vi "UHR-Fleezers Control (host) - Avogadro v1.vi"() -> ()   [LabVIEW 2014] (continued)
        n65 = event-data() -> ()  [unwired: 1 in, 5 out]
        n66 = Build Array("Set Position 1", "Set Position 2", "Set Position 3", "Set Position 4", "Set Position 5", "Set Position 6") -> (w238:bool[])
        n67 = Boolean Array To Number(Boolean array=w238) -> (number=w237:u32)
        n68 = Logarithm Base 2(1:w237) -> (0:w229:dbl)
        n69 = call "Read Stage Position.vi"("error in"=w239, "VISA resource name in"=w240) -> ("Current Position"=w244:cluster{dbl, dbl, dbl}, "error out"=w243:errorcluster)  [unwired: 2 out]
        n70 = Decrement(x="Position") -> (x-1=w227:dbl)
        n71 = Greater Or Equal?(x=w229, y=0.0) -> (x >= y?=w230:bool)
        n72 = Cluster To Array(cluster=w244) -> (array=w241:dbl[])
        n73 = Select(t=w229, s=w230, f=w227) -> (s? t:f=w226:dbl)
        n74 = local write "Stage Control Serial Error"(w243) -> ()
        n75 = Increment(x=w226) -> (x+1=w225:dbl)
        n76 = Build Array (concatenate)(w225, w241) -> (w224:dbl[])
        n77 = Replace Array Subset(array="Saved Stage Positions", new element=w224, index (row)=w226) -> (w242:dbl[][])  [unwired: 1 in]
        n78 = local write "Saved Stage Positions"(w242) -> ()
      }
      event Menu Selection (User) {
        n79 = event-data() -> ("ItemTag"=w249:string)  [unwired: 1 in, 6 out]
        n80 = case shown="\"Z\"" w249 {
          tunnel: w248 -> [_ w251 w256 _]
          tunnel: w247 -> [_ w250 w254 _]
          frame "False", Default {
          }
          frame "XY" {
            n81 = call "start_stage_trackball.vi"("Enum"=T38."Trackball XY", "error in (no error)"=w250, "Stage Controller port"=w251) -> ("error out"=w253:errorcluster)  [unwired: 1 out]
            n82 = property on="Stage Control Serial Error" class="Clust (strict)"("Val(Sgnl)"=w253) -> ()  [unwired: 2 in, 2 out]
          }
          frame "Z" {
            n83 = call "start_stage_trackball.vi"("Enum"=T38."Trackball Z", "error in (no error)"=w254, "Stage Controller port"=w256) -> ("error out"=w255:errorcluster)  [unwired: 1 out]
            n84 = property on="Stage Control Serial Error" class="Clust (strict)"("Val(Sgnl)"=w255) -> ()  [unwired: 2 in, 2 out]
          }
          frame "True" {
          }
        }
      }
      event "Move to Position": Value Change {
        n85 = event-data() -> ()  [unwired: 1 in, 5 out]
        n86 = flat-sequence {
          tunnel: w259 -> [w263]
          tunnel: w258 -> [w262]
          frame #0 {
            n87 = local read "Saved Stage Positions"() -> (w265:dbl[][])
            n88 = local read "Position"() -> (w264:dbl)
            n89 = local write "Stage Moving"(TRUE ("Stage Moving")) -> ()
            n90 = call "move to saved stage position.vi"("error in"=w262, "Stage VISA resource name in"=w263, "Position"=w264, "Saved Stage Positions"=w265) -> ("error out"=w261:errorcluster)  [unwired: 1 out]
            n91 = local write "Stage Control Serial Error"(w261) -> ()
          }
          frame #1 {
            n92 = call <vilib>:"Beep.vi"() -> ()  [unwired: 3 in, 9 out]
            n93 = local write "Stage Moving"(FALSE ("Stage Moving")) -> ()
          }
        }
      }
      event "Move Cap. 1 (DNA Bottom)": Value Change {
        n94 = event-data() -> ()  [unwired: 1 in, 5 out]
        n95 = local write "Move Cap. 1 (DNA Bottom)"(FALSE ("Move Cap. 1 (DNA Right)")) -> ()
        n96 = flat-sequence {
          tunnel: w271 -> [w274]
          tunnel: w272 -> [w275]
          tunnel: [w275] -> w269
          tunnel: [w274] -> w268
          tunnel: w269 -> [w277]
          tunnel: w268 -> [w276]
          frame #0 {
            n97 = property on="Sample Channel\nFlow" class="Bool (strict)"("Val(Sgnl)"="Cap 1 Samp Flow ON") -> ()  [unwired: 2 in, 2 out]
          }
          frame #1 {
            n98 = local read "Saved Stage Positions"() -> (w287:dbl[][])
            n99 = local write "Stage Moving"(TRUE ("Stage Moving")) -> ()
            n100 = Array Subset(array=w287, index (row)=0 ("index"), length (row)=1 ("length"), index (col)=1 ("index"), length (col)=3 ("length")) -> (w284:dbl[][])
            n101 = Reshape Array(w284, 3 ("dimension size")) -> (w282:dbl[])
            n102 = Array To Cluster(array=w282) -> (cluster=w281:cluster{"[0]":dbl, "[1]":dbl, "[2]":dbl})
            n103 = call "Set Stage Position.vi"("Position"=w281, "error in"=w276, "VISA resource name in"=w277) -> ("error out"=w280:errorcluster)  [unwired: 2 out]
            n104 = local write "Stage Control Serial Error"(w280) -> ()
          }
          frame #2 {
            n105 = local write "Stage Moving"(FALSE ("Stage Moving")) -> ()
            n106 = case shown="True" "Cap 1 Flow ON" {
              frame False {
              }
              frame True {
                n107 = property on="Inject Pump 1" class="Bool (strict)"("Val(Sgnl)"=TRUE ("Value (Signaling)")) -> ()  [unwired: 2 in, 2 out]
              }
            }
            n108 = call <vilib>:"Beep.vi"() -> ()  [unwired: 3 in, 9 out]
          }
          frame #3 {
            n109 = property on="Sample Channel\nFlow" class="Bool (strict)"("Val(Sgnl)"=FALSE ("Value (Signaling)")) -> ()  [unwired: 2 in, 2 out]
            n110 = local read "Cap. 2 BD T1?\n(ADig T1, DNA T2)"() -> (w294:bool)
            n111 = case shown="True" w294 {
              tunnel: "Cap 1 T ON" -> [w296 w297]
              frame False {
                n112 = property on="Trap 1 (ON/OFF)" class="Bool (strict)"("Val(Sgnl)"=w296) -> ()  [unwired: 2 in, 2 out]
              }
              frame True {
                n113 = property on="Trap 2 (ON/OFF)" class="Bool (strict)"("Val(Sgnl)"=w297) -> ()  [unwired: 2 in, 2 out]
              }
            }
            n114 = property on="Get bead 2" class="Bool (strict)"("Key Focus"=TRUE) -> ()  [unwired: 2 in, 2 out]
          }
        }
      }
      event "Move Cap. 2 (ADig Top)": Value Change {
        n115 = event-data() -> ()  [unwired: 1 in, 5 out]
        n116 = local write "Move Cap. 2 (ADig Top)"(FALSE ("Move Cap. 2 (ADig Left)")) -> ()
        n117 = flat-sequence {
          tunnel: w301 -> [w304]
          tunnel: w302 -> [w305]
          tunnel: [w305] -> w299
          tunnel: [w304] -> w298
          tunnel: w299 -> [w308]
          tunnel: w298 -> [w307]
          frame #0 {
            n118 = property on="Sample Channel\nFlow" class="Bool (strict)"("Val(Sgnl)"="Cap 2 Samp Flow ON") -> ()  [unwired: 2 in, 2 out]
          }
          frame #1 {
            w306 = FALSE ("Value (Signaling)")
            n119 = local read "Saved Stage Positions"() -> (w318:dbl[][])
            n120 = local write "Stage Moving"(TRUE ("Stage Moving")) -> ()
            n121 = Array Subset(array=w318, index (row)=1 ("index"), length (row)=1 ("length"), index (col)=1 ("index"), length (col)=3 ("length")) -> (w315:dbl[][])
            n122 = Reshape Array(w315, 3 ("dimension size")) -> (w313:dbl[])
            n123 = property on="Trap 1 (ON/OFF)" class="Bool (strict)"("Val(Sgnl)"=w306) -> ()  [unwired: 2 in, 2 out]
            n124 = property on="Trap 1 (ON/OFF)" class="Bool (strict)"("Val(Sgnl)"=w306) -> ()  [unwired: 2 in, 2 out]
            n125 = Array To Cluster(array=w313) -> (cluster=w312:cluster{"[0]":dbl, "[1]":dbl, "[2]":dbl})
            n126 = call "Set Stage Position.vi"("Position"=w312, "error in"=w307, "VISA resource name in"=w308) -> ("error out"=w311:errorcluster)  [unwired: 2 out]
            n127 = local write "Stage Control Serial Error"(w311) -> ()
          }
          frame #2 {
            n128 = local write "Stage Moving"(FALSE ("Stage Moving")) -> ()
            n129 = call <vilib>:"Beep.vi"() -> ()  [unwired: 3 in, 9 out]
            n130 = case shown="True" "Cap 2 Flow ON" {
              frame False {
              }
              frame True {
                n131 = property on="Inject Pump 3" class="Bool (strict)"("Val(Sgnl)"=TRUE ("Value (Signaling)")) -> ()  [unwired: 2 in, 2 out]
              }
            }
          }
          frame #3 {
            n132 = property on="Sample Channel\nFlow" class="Bool (strict)"("Val(Sgnl)"=FALSE ("Value (Signaling)")) -> ()  [unwired: 2 in, 2 out]
            n133 = case shown="False" "Cap. 2 BD T1?\n(ADig T1, DNA T2)" {
              tunnel: "Cap 2 T ON" -> [w327 w328]
              frame False {
                n134 = property on="Trap 2 (ON/OFF)" class="Bool (strict)"("Val(Sgnl)"=w327) -> ()  [unwired: 2 in, 2 out]
              }
              frame True {
                n135 = property on="Trap 1 (ON/OFF)" class="Bool (strict)"("Val(Sgnl)"=w328) -> ()  [unwired: 2 in, 2 out]
              }
            }
            n136 = property on="Get bead 3" class="Bool (strict)"("Key Focus"=TRUE) -> ()  [unwired: 2 in, 2 out]
          }
        }
      }
      event "Send string\nto Blue Laser": Value Change {
        n137 = event-data() -> ()  [unwired: 1 in, 5 out]
        n138 = flat-sequence {
          tunnel: w329 -> [w330]
          frame #0 {
            n139 = call "serial write macro.vi"("String"="command string", "Delay (ms)"="Delay (ms)", "VISA resource name"=w330) -> ("read buffer"=→"read blue buffer":string, "error out"=→"Blue Error Out":errorcluster)  [unwired: 1 out]
            "command string sent" <- "command string"
          }
          frame #1 {
            n140 = local write "Send string\nto Blue Laser"(FALSE ("Send string")) -> ()
          }
        }
      }
      event "Get Blue Laser State": Value Change {
        n141 = event-data() -> ()  [unwired: 1 in, 5 out]
        n142 = local read "Delay (ms)"() -> (w337:i32)
        n143 = flat-sequence {
          tunnel: w337 -> [w345]
          tunnel: w336 -> [w348]
          tunnel: [w346] -> w341
          tunnel: [w345] -> w340
          tunnel: [w355] -> w339
          tunnel: [w352] -> w338
          tunnel: w341 -> [w353]
          tunnel: w340 -> [w352]
          tunnel: w339 -> [w361]
          tunnel: w338 -> [w359]
          frame #0 {
            w343 = "l?"
            n144 = local write "command string sent"(w343) -> ()
            n145 = call "serial write macro.vi"("String"=w343, "Delay (ms)"=w345, "VISA resource name"=w348) -> ("read buffer"=w344:string, "VISA resource name out"=w346:refnum<visa-resource-name>)  [unwired: 1 out]
            n146 = Decimal String To Number(string=w344) -> (number=w347:i32)  [unwired: 2 in, 1 out]
            n147 = Not Equal To 0?(x=w347) -> (x != 0?=→"Laser On":bool)
            n148 = local write "read blue buffer"(w344) -> ()
          }
          frame #1 {
            w350 = "games?" ("String")
            n149 = local write "command string sent"(w350) -> ()
            n150 = call "serial write macro.vi"("String"=w350, "Delay (ms)"=w352, "VISA resource name"=w353) -> ("read buffer"=w351:string, "VISA resource name out"=w355:refnum<visa-resource-name>)  [unwired: 1 out]
            n151 = Decimal String To Number(string=w351) -> (number=w354:i32)  [unwired: 2 in, 1 out]
            n152 = local write "read blue buffer"(w351) -> ()
            n153 = Not Equal To 0?(x=w354) -> (x != 0?=→"Analog Modulation":bool)
          }
          frame #2 {
            w357 = "gdmes?" ("String")
            n154 = local write "command string sent"(w357) -> ()
            n155 = call "serial write macro.vi"("String"=w357, "Delay (ms)"=w359, "VISA resource name"=w361) -> ("read buffer"=w358:string)  [unwired: 2 out]
            n156 = Decimal String To Number(string=w358) -> (number=w360:i32)  [unwired: 2 in, 1 out]
            n157 = Not Equal To 0?(x=w360) -> (x != 0?=→"Digital Modulation":bool)
            n158 = local write "read blue buffer"(w358) -> ()
          }
          frame #3 {
            n159 = local write "Get Blue Laser State"(FALSE) -> ()
          }
        }
      }
      event "Blue Laser Power (mW)\n(Constant Power Mode)", "Blue Laser Modulation\nPower (mW)": Value Change {
        n160 = event-data() -> ()  [unwired: 1 in, 5 out]
        n161 = flat-sequence {
          tunnel: w364 -> [w370]
          tunnel: [w368] -> w363
          tunnel: w363 -> [w377]
          frame #0 {
            n162 = local read "Delay (ms)"() -> (w369:i32)
            n163 = Concatenate Strings("slmp " ("string"), "Blue Laser Modulation\nPower (mW)") -> (w365:string)
            n164 = call "serial write macro.vi"("String"=w365, "Delay (ms)"=w369, "VISA resource name"=w370) -> ("read buffer"=w366:string, "error out"=w367:errorcluster, "VISA resource name out"=w368:refnum<visa-resource-name>)
            n165 = local write "command string sent"(w365) -> ()
            n166 = local write "read blue buffer"(w366) -> ()
            n167 = local write "Blue Error Out"(w367) -> ()
          }
          frame #1 {
            n168 = local read "Delay (ms)"() -> (w376:i32)
            n169 = Concatenate Strings("p " ("string"), "Blue Laser Power (mW)\n(Constant Power Mode)") -> (w373:string)
            n170 = call "serial write macro.vi"("String"=w373, "Delay (ms)"=w376, "VISA resource name"=w377) -> ("read buffer"=w374:string, "error out"=w375:errorcluster)  [unwired: 1 out]
            n171 = local write "command string sent"(w373) -> ()
            n172 = local write "read blue buffer"(w374) -> ()
            n173 = local write "Blue Error Out"(w375) -> ()
          }
        }
      }
      event "Laser interlacing mode", "Blue Laser Modulation Mode", "Blue Laser ON": Value Change {
        n174 = event-data() -> ()  [unwired: 1 in, 5 out]
        n175 = flat-sequence {
          tunnel: w383 -> [w388]
          tunnel: [w387] -> w380
          tunnel: [w393] -> w382
          tunnel: w380 -> [w396]
          tunnel: w382 -> [w408]
          tunnel: [w402] -> w381
          tunnel: w381 -> [w415]
          frame #0 {
            n176 = local read "Blue Laser ON"() -> (w385:bool)
            n177 = local read "Delay (ms)"() -> (w386:i32)
            n178 = case shown="False" w385 {
              tunnel: ["l0" "l1"] -> w384
              frame False {
              }
              frame True {
              }
            }
            n179 = call "serial write macro.vi"("String"=w384, "Delay (ms)"=w386, "VISA resource name"=w388) -> ("error out"=w389:errorcluster, "VISA resource name out"=w387:refnum<visa-resource-name>)  [unwired: 1 out]
            n180 = local write "Blue Error Out"(w389) -> ()
          }
          frame #1 {
            n181 = local read "Laser interlacing mode"() -> (w398:enum32{"Laser ON", "Laser OFF", "Interlace"})
            n182 = case shown="\"Laser ON\"" w398 {
              tunnel: ["cp" "em" "l0"] -> w392
              frame "Laser ON" {
              }
              frame "Interlace" {
              }
              frame "Laser OFF", Default {
              }
            }
            n183 = local read "Delay (ms)"() -> (w397:i32)
            n184 = call "serial write macro.vi"("String"=w392, "Delay (ms)"=w397, "VISA resource name"=w396) -> ("read buffer"=w394:string, "error out"=w395:errorcluster, "VISA resource name out"=w393:refnum<visa-resource-name>)
            n185 = local write "command string sent"(w392) -> ()
            n186 = local write "read blue buffer"(w394) -> ()
            n187 = local write "Blue Error Out"(w395) -> ()
          }
          frame #2 {
            n188 = case shown="\"Analog Modulation\"" "Blue Laser Modulation Mode" {
              tunnel: ["sdmes 0" "sdmes 1" "sdmes 1"] -> w403
              frame "Analog Modulation" {
              }
              frame "Digital + Analog Modulation" {
              }
              frame "Digital Modulation", Default {
              }
            }
            n189 = local read "Delay (ms)"() -> (w406:i32)
            n190 = call "serial write macro.vi"("String"=w403, "Delay (ms)"=w406, "VISA resource name"=w408) -> ("read buffer"=w404:string, "error out"=w405:errorcluster, "VISA resource name out"=w402:refnum<visa-resource-name>)
            n191 = local write "command string sent"(w403) -> ()
            n192 = local write "read blue buffer"(w404) -> ()
            n193 = local write "Blue Error Out"(w405) -> ()
          }
          frame #3 {
            n194 = local read "Blue Laser Modulation Mode"() -> (w417:string)
            n195 = case shown="\"Digital Modulation\", Default" w417 {
              tunnel: ["sames 1" "sames 1" "sames 0"] -> w413
              frame "Analog Modulation" {
              }
              frame "Digital + Analog Modulation" {
              }
              frame "Digital Modulation", Default {
              }
            }
            n196 = local read "Delay (ms)"() -> (w416:i32)
            n197 = local write "command string sent"(w413) -> ()
            n198 = call "serial write macro.vi"("String"=w413, "Delay (ms)"=w416, "VISA resource name"=w415) -> ("read buffer"=w414:string, "error out"=w412:errorcluster)  [unwired: 1 out]
            n199 = local write "read blue buffer"(w414) -> ()
            n200 = local write "Blue Error Out"(w412) -> ()
          }
        }
      }
      event "Read Harvard": Value Change {
        n201 = event-data() -> ()  [unwired: 1 in, 5 out]
        n202 = Concatenate Strings("write buffer", "\r") -> (w425:string)
        n203 = VISA Write(VISA resource name=w423, write buffer=w425, error in (no error)=w422) -> (VISA resource name out=w434:refnum<visa-resource-name>, error out=w433:errorcluster)  [unwired: 1 out]
        n204 = stacked-sequence {
          tunnel: [w437] -> w432
          tunnel: w434 -> [w437]
          tunnel: w433 -> [w436]
          tunnel: [w436] -> w427
          frame #0 {
            n205 = Wait (ms)(milliseconds to wait=50) -> ()  [unwired: 1 out]
          }
        }
        n206 = property class="Instr"(reference=w432, error in=w427) -> (reference out=w431:refnum<visa-resource-name>, error out=w429:errorcluster, "Serial Settings:Number of Bytes at Serial Port"=w430:u32)
        "Serial Settings:Number of Bytes at Serial Port" <- w430
        n207 = VISA Read(VISA resource name=w431, byte count=w430, error in (no error)=w429) -> (read buffer=w428:string)  [unwired: 3 out]
        "read buffer" <- w428
        n208 = Fract/Exp String To Number(string=w428) -> ()  [unwired: 5 out]
      }
      event "+z", "-z": Value Change {
        n209 = event-data() -> ()  [unwired: 1 in, 5 out]
        n210 = flat-sequence {
          tunnel: w438 -> [w460]
          tunnel: w439 -> [w440]
          frame #0 {
            n211 = call "Read Stage Position.vi"("error in"=w460, "VISA resource name in"=w440) -> ("Current Position"=w445:cluster{dbl, dbl, dbl}, "error out"=w458:errorcluster, "VISA resource name out"=w459:refnum<visa-resource-name>)  [unwired: 1 out]
            n212 = local read "Saved Stage Positions"() -> (w469:dbl[][])
            n213 = Divide(x="z nudge increment (um)", y=1000.0) -> (x/y=w457:dbl)
            n214 = Boolean To (0,1)(Boolean="+z") -> (0, 1=w449:i16)
            n215 = Boolean To (0,1)(Boolean="-z") -> (0, 1=w450:i16)
            n216 = Array Subset(array=w469, index (row)=1 ("index"), length (row)=1 ("length"), index (col)=1 ("index"), length (col)=3 ("length")) -> (w466:dbl[][])
            n217 = Multiply(x=w449, y=w457) -> (x*y=w453:dbl)
            n218 = Multiply(x=w450, y=w457) -> (x*y=w451:dbl)
            n219 = Unbundle(w445) -> (w443:dbl, w442:dbl, w446:dbl)
            n220 = Negate(x=w451) -> (-x=w452:dbl)
            n221 = Reshape Array(w466, 3 ("dimension size")) -> (w464:dbl[])
            n222 = Add(x=w453, y=w452) -> (x+y=w454:dbl)
            n223 = Array To Cluster(array=w464) -> ()  [unwired: 1 out]
            n224 = Add(x=w454, y=w446) -> (x+y=w444:dbl)
            n225 = Bundle(cluster=w445, w443, w442, w444) -> (w441:cluster{dbl, dbl, dbl})
            n226 = call "Set Stage Position.vi"("Position"=w441, "error in"=w458, "VISA resource name in"=w459) -> ("error out"=w463:errorcluster)  [unwired: 2 out]
            n227 = local write "Stage Moving"(TRUE ("Stage Moving")) -> ()
            n228 = local write "Stage Control Serial Error"(w463) -> ()
          }
          frame #1 {
            n229 = local write "Stage Moving"(FALSE ("Stage Moving")) -> ()
          }
        }
      }
      event "-y", "+y": Value Change {
        n230 = event-data() -> ()  [unwired: 1 in, 5 out]
        n231 = flat-sequence {
          tunnel: w472 -> [w496]
          tunnel: w473 -> [w479]
          frame #0 {
            n232 = call "Read Stage Position.vi"("error in"=w496, "VISA resource name in"=w479) -> ("Current Position"=w482:cluster{dbl, dbl, dbl}, "error out"=w494:errorcluster, "VISA resource name out"=w495:refnum<visa-resource-name>)  [unwired: 1 out]
            n233 = Divide(x="y nudge increment (um", y=1000.0) -> (x/y=w493:dbl)
            n234 = Boolean To (0,1)(Boolean="+y") -> (0, 1=w485:i16)
            n235 = Boolean To (0,1)(Boolean="-y") -> (0, 1=w486:i16)
            n236 = Multiply(x=w485, y=w493) -> (x*y=w489:dbl)
            n237 = Multiply(x=w486, y=w493) -> (x*y=w487:dbl)
            n238 = Unbundle(w482) -> (w481:dbl, w476:dbl, w478:dbl)
            n239 = Negate(x=w487) -> (-x=w488:dbl)
            n240 = Add(x=w489, y=w488) -> (x+y=w490:dbl)
            n241 = Add(x=w490, y=w476) -> (x+y=w477:dbl)
            n242 = Bundle(cluster=w482, w481, w477, w478) -> (w480:cluster{dbl, dbl, dbl})
            n243 = call "Set Stage Position.vi"("Position"=w480, "error in"=w494, "VISA resource name in"=w495) -> ("error out"=w475:errorcluster)  [unwired: 2 out]
            n244 = local write "Stage Control Serial Error"(w475) -> ()
            n245 = local write "Stage Moving"(TRUE ("Stage Moving")) -> ()
          }
          frame #1 {
            n246 = local write "Stage Moving"(FALSE ("Stage Moving")) -> ()
          }
        }
      }
      event "-x", "+x": Value Change {
        n247 = event-data() -> ()  [unwired: 1 in, 5 out]
        n248 = flat-sequence {
          tunnel: w498 -> [w522]
          tunnel: w499 -> [w506]
          frame #0 {
            n249 = call "Read Stage Position.vi"("error in"=w522, "VISA resource name in"=w506) -> ("Current Position"=w508:cluster{dbl, dbl, dbl}, "error out"=w520:errorcluster, "VISA resource name out"=w521:refnum<visa-resource-name>)  [unwired: 1 out]
            n250 = Divide(x="x nudge increment (um)", y=1000.0) -> (x/y=w519:dbl)
            n251 = Boolean To (0,1)(Boolean="+x") -> (0, 1=w511:i16)
            n252 = Boolean To (0,1)(Boolean="-x") -> (0, 1=w512:i16)
            n253 = Multiply(x=w511, y=w519) -> (x*y=w515:dbl)
            n254 = Multiply(x=w512, y=w519) -> (x*y=w513:dbl)
            n255 = Unbundle(w508) -> (w500:dbl, w502:dbl, w505:dbl)
            n256 = Negate(x=w513) -> (-x=w514:dbl)
            n257 = Add(x=w515, y=w514) -> (x+y=w516:dbl)
            n258 = Add(x=w516, y=w500) -> (x+y=w501:dbl)
            n259 = Bundle(cluster=w508, w501, w502, w505) -> (w507:cluster{dbl, dbl, dbl})
            n260 = call "Set Stage Position.vi"("Position"=w507, "error in"=w520, "VISA resource name in"=w521) -> ("error out"=w503:errorcluster)  [unwired: 2 out]
            n261 = local write "Stage Control Serial Error"(w503) -> ()
            n262 = local write "Stage Moving"(TRUE ("Stage Moving")) -> ()
          }
          frame #1 {
            n263 = local write "Stage Moving"(FALSE ("Stage Moving")) -> ()
          }
        }
      }
      event "Cal/Data Acq. Spot": Value Change {
        # "03-01-2018 Changed by RG to incorporate offset measurements at multiple \npositions of the piezo mirror"
        # "Disabled by Ronen - we have our own way of controlling the location of calibration."
        n264 = event-data() -> ()  [unwired: 1 in, 5 out]
        n265 = flat-sequence {
          tunnel: w531 -> [w535]
          tunnel: w532 -> [w536]
          tunnel: [w536] -> w528
          tunnel: [w535] -> w527
          tunnel: w528 -> [w539]
          tunnel: w527 -> [w538]
          tunnel: ["Cal @ (MHz)"] -> w525
          tunnel: [w547] -> w529
          tunnel: w525 -> [w547]
          tunnel: w529 -> [w560]
          tunnel: ["W/ Offset 1"] -> w526
          tunnel: w524 -> [w558]
          tunnel: w529 -> [w596]
          tunnel: w526 -> [w594]
          frame #0 {
            n266 = property on="Sample Channel\nFlow" class="Bool (strict)"("Val(Sgnl)"="Daq spot flow on") -> ()  [unwired: 2 in, 2 out]
            n267 = Wait (ms)(milliseconds to wait=u32 250) -> ()  [unwired: 1 out]
          }
          frame #1 {
            n268 = disable-structure shown="Disabled" {
              disable-tunnel: w539 -> [w544 _]
              disable-tunnel: w538 -> [w543 _]
              frame Disabled {
                n269 = local read "Saved Stage Positions"() -> (w541:dbl[][])
                n270 = call "move to saved stage position.vi"("error in"=w543, "Stage VISA resource name in"=w544, "Position"="Cal Stage Position", "Saved Stage Positions"=w541) -> ("error out"=w542:errorcluster)  [unwired: 1 out]
                n271 = local write "Stage Control Serial Error"(w542) -> ()
              }
              frame Enabled {
              }
            }
            n272 = property on="Trap Delta (MHz)" class="DigNum (strict)"("Val(Sgnl)"="Cal @ (MHz)") -> ()  [unwired: 2 in, 2 out]
            n273 = local write "Stage Moving"(TRUE ("Stage Moving")) -> ()
          }
          frame #2 {
            n274 = local write "Stage Moving"(FALSE ("Stage Moving")) -> ()
            n275 = property on="Sample Channel\nFlow" class="Bool (strict)"("Val(Sgnl)"="Flow ON during cal?") -> ()  [unwired: 2 in, 2 out]
            n276 = call <vilib>:"Beep.vi"() -> ()  [unwired: 3 in, 9 out]
          }
          frame #3 {
            n277 = Wait (ms)(milliseconds to wait=u32 1000) -> ()  [unwired: 1 out]
          }
          frame #4 {
            n278 = case shown="False" "Active cal after cal?" {
              frame False {
              }
              frame True {
                n279 = local write "Active Cal"(TRUE ("Active Cal")) -> ()
                n280 = Wait (ms)(milliseconds to wait=u32 8000) -> ()  [unwired: 1 out]
              }
            }
          }
          frame #5 {
            n281 = property on="Save Calibration" class="Bool (strict)"("Val(Sgnl)"=TRUE ("Value (Signaling)")) -> ()  [unwired: 2 in, 2 out]
          }
          frame #6 {
            n282 = Wait (ms)(milliseconds to wait=u32 2000) -> ()  [unwired: 1 out]
          }
          frame #7 {
            # "Check to see if \nsaving done"
            n283 = while {
              stop <- w555 stop-if-true
              n284 = local read "Saving..."() -> (w556:bool)
              n285 = Wait (ms)(milliseconds to wait=u32 100) -> ()  [unwired: 1 out]
              n286 = Not(x=w556) -> (.not. x?=w555:bool)
            }
          }
          frame #8 {
            n287 = case shown="True" "W/ Offset 1" {
              tunnel: w560 -> [_ w562]
              tunnel: w558 -> [_ w561]
              frame False {
              }
              frame True {
                n288 = stacked-sequence {
                  tunnel: w562 -> [_ _ _ _ _ _ _ _ _ w593]
                  tunnel: w561 -> [_ _ _ _ w571 _ _ _ _ w591]
                  frame #0 {
                    n289 = property on="Trap Delta (MHz)" class="DigNum (strict)"("Val(Sgnl)"="Offset 1 Start (MHz)") -> ()  [unwired: 2 in, 2 out]
                    n290 = Replace Array Subset(array=u32[] [0] ("Index Values"), new element="Offset 1 Set", index=0) -> (w564:u32[])
                    n291 = property on="Saved AOD Raster Scan Parameter Sets" class="Arr (strict)"("Index Values"=w564) -> ()  [unwired: 2 in, 2 out]
                    n292 = property on="manual raster set" class="Ring (strict)"("Value"="Offset 1 Set") -> ()  [unwired: 2 in, 2 out]
                  }
                  frame #1 {
                    n293 = Wait (ms)(milliseconds to wait=u32 200) -> ()  [unwired: 1 out]
                  }
                  frame #2 {
                    n294 = property on="Load parameters" class="Bool (strict)"("Val(Sgnl)"=TRUE ("Value (Signaling)")) -> ()  [unwired: 2 in, 2 out]
                  }
                  frame #3 {
                    n295 = Wait (ms)(milliseconds to wait=u32 200) -> ()  [unwired: 1 out]
                  }
                  frame #4 {
                    n296 = case shown="True" "Multiple-MCL offset?" {
                      tunnel: w571 -> [_ w580]
                      frame False {
                      }
                      frame True {
                        n297 = call "Make Trap3 position array.vi"("MCL offset scanning range (V)"="MCL offset scanning range (V)") -> ("Scan increment"=w575:u64, "Min Y"=w576:u64, "Min X"=w577:u64, "X Data points"=w578:u64, "Y data points"=w579:u64)
                        n298 = Multiply(x=w579, y=w578) -> (x*y=w573:u64)
                        n299 = xnode "Read/Write Control"("FPGA VI Reference In"=w580, "Number of scans"=w573, "Piezo offset Y points"=w579, "Piezo offset X points"=w578, "Piezo offset Xmin"=w577, "Piezo Offset Ymin"=w576, "Piezo Offset Increment"=w575, "Multiple trap 3 position offset  file"=TRUE) -> ()  [unwired: 1 in, 2 out]
                        n300 = property on="Number of F/B Scans (AOD)" class="DigNum (strict)"("Val(Sgnl)"=w573) -> ()  [unwired: 2 in, 2 out]
                      }
                    }
                  }
                  frame #5 {
                    n301 = Wait (ms)(milliseconds to wait=u32 200) -> ()  [unwired: 1 out]
                  }
                  frame #6 {
                    n302 = property on="Trap Raster Scan" class="Bool (strict)"("Val(Sgnl)"=TRUE ("Value (Signaling)")) -> ()  [unwired: 2 in, 2 out]
                  }
                  frame #7 {
                    n303 = Wait (ms)(milliseconds to wait=u32 2000) -> ()  [unwired: 1 out]
                  }
                  frame #8 {
                    n304 = while {
                      stop <- w588 stop-if-true
                      n305 = local read "Raster Scanning..."() -> (w590:bool)
                      n306 = local read "Saving..."() -> (w586:bool)
                      n307 = Wait (ms)(milliseconds to wait=u32 100) -> ()  [unwired: 1 out]
                      n308 = Not(x=w586) -> (.not. x?=w585:bool)
                      n309 = Not(x=w590) -> (.not. x?=w587:bool)
                      n310 = And(x=w587, y=w585) -> (x .and. y?=w588:bool)
                    }
                  }
                  frame #9 {
                    n311 = property on="Trap Delta (MHz)" class="DigNum (strict)"("Val(Sgnl)"=w593) -> ()  [unwired: 2 in, 2 out]
                    n312 = xnode "Read/Write Control"("FPGA VI Reference In"=w591, "Multiple trap 3 position offset  file"=FALSE) -> ()  [unwired: 1 in, 2 out]
                  }
                }
              }
            }
          }
          frame #9 {
            n313 = local read "Save ave N"() -> (w595:dbl)
            n314 = case shown="False" "W/ Offset 2" {
              tunnel: w596 -> [_ w603]
              tunnel: w595 -> [_ w602]
              tunnel: w594 -> [w598 _]
              frame False {
                n315 = case shown="False" w598 {
                  frame False {
                    n316 = Multiply(x="Cal read wait (s)", y=u32 1000 ("milliseconds to wait")) -> (x*y=w600:u32)
                    n317 = Wait (ms)(milliseconds to wait=w600) -> ()  [unwired: 1 out]
                  }
                  frame True {
                  }
                }
              }
              frame True {
                n318 = stacked-sequence {
                  tunnel: w603 -> [_ _ _ _ _ _ _ _ _ w624 _ _]
                  tunnel: w602 -> [_ _ _ _ _ _ _ _ _ w622 _ _]
                  frame #0 {
                    n319 = property on="Save ave N" class="DigNum (strict)"("Val(Sgnl)"=1.0 ("Value (Signaling)")) -> ()  [unwired: 2 in, 2 out]
                  }
                  frame #1 {
                    n320 = Wait (ms)(milliseconds to wait=u32 500) -> ()  [unwired: 1 out]
                  }
                  frame #2 {
                    n321 = property on="Trap Delta (MHz)" class="DigNum (strict)"("Val(Sgnl)"="Offset 2 Start (MHz)") -> ()  [unwired: 2 in, 2 out]
                    n322 = Replace Array Subset(array=u32[] [0] ("Index Values"), new element="Offset 2 Set", index=0) -> (w608:u32[])
                    n323 = property on="Saved AOD Raster Scan Parameter Sets" class="Arr (strict)"("Index Values"=w608) -> ()  [unwired: 2 in, 2 out]
                  }
                  frame #3 {
                    n324 = Wait (ms)(milliseconds to wait=u32 500) -> ()  [unwired: 1 out]
                  }
                  frame #4 {
                    n325 = property on="Load parameters" class="Bool (strict)"("Val(Sgnl)"=TRUE ("Value (Signaling)")) -> ()  [unwired: 2 in, 2 out]
                  }
                  frame #5 {
                    n326 = Wait (ms)(milliseconds to wait=u32 500) -> ()  [unwired: 1 out]
                  }
                  frame #6 {
                    n327 = property on="Trap Raster Scan" class="Bool (strict)"("Val(Sgnl)"=TRUE ("Value (Signaling)")) -> ()  [unwired: 2 in, 2 out]
                  }
                  frame #7 {
                    n328 = Wait (ms)(milliseconds to wait=u32 2000) -> ()  [unwired: 1 out]
                  }
                  frame #8 {
                    n329 = while {
                      stop <- w617 stop-if-true
                      n330 = local read "Raster Scanning..."() -> (w620:bool)
                      n331 = local read "Saving..."() -> (w618:bool)
                      n332 = Wait (ms)(milliseconds to wait=u32 100) -> ()  [unwired: 1 out]
                      n333 = Not(x=w618) -> (.not. x?=w616:bool)
                      n334 = Not(x=w620) -> (.not. x?=w619:bool)
                      n335 = And(x=w619, y=w616) -> (x .and. y?=w617:bool)
                    }
                  }
                  frame #9 {
                    n336 = property on="Trap Delta (MHz)" class="DigNum (strict)"("Val(Sgnl)"=w624) -> ()  [unwired: 2 in, 2 out]
                    n337 = property on="Saved AOD Raster Scan Parameter Sets" class="Arr (strict)"("Index Values"=u32[] [0]) -> ()  [unwired: 2 in, 2 out]
                    n338 = property on="Save ave N" class="DigNum (strict)"("Val(Sgnl)"=w622) -> ()  [unwired: 2 in, 2 out]
                  }
                  frame #10 {
                    n339 = Wait (ms)(milliseconds to wait=u32 500) -> ()  [unwired: 1 out]
                  }
                  frame #11 {
                    n340 = property on="Load parameters" class="Bool (strict)"("Val(Sgnl)"=TRUE ("Value (Signaling)")) -> ()  [unwired: 2 in, 2 out]
                  }
                }
              }
            }
          }
          frame #10 {
            n341 = property on="Read Cal" class="Bool (strict)"("Val(Sgnl)"=TRUE ("Value (Signaling)")) -> ()  [unwired: 2 in, 2 out]
          }
          frame #11 {
            n342 = Wait (ms)(milliseconds to wait=u32 1000) -> ()  [unwired: 1 out]
          }
          frame #12 {
            n343 = property on="Fish for Tether" class="Bool (strict)"("Val(Sgnl)"="Fish after cal?") -> ()  [unwired: 2 in, 2 out]
          }
        }
        n344 = local write "Cal/Data Acq. Spot"(FALSE ("Cal/Data Acq. Spot")) -> ()
      }
      event "Dump Beads": Value Change {
        n345 = event-data() -> ()  [unwired: 1 in, 5 out]
        n346 = flat-sequence {
          tunnel: ["Dump spot flow on?"] -> w630
          tunnel: [w641] -> w631
          tunnel: w630 -> [w641]
          tunnel: w634 -> [w646]
          tunnel: w633 -> [w645]
          tunnel: [w643] -> w632
          tunnel: w631 -> [w643]
          tunnel: w632 -> [w656]
          frame #0 {
            w635 = FALSE ("Value (Signaling)")
            n347 = local read "Saving..."() -> (w637:bool)
            n348 = local write "Dump Beads"(FALSE ("Dump Beads")) -> ()
            n349 = property on="Inject Pump 3" class="Bool (strict)"("Val(Sgnl)"=w635) -> ()  [unwired: 2 in, 2 out]
            n350 = property on="Inject Pump 1" class="Bool (strict)"("Val(Sgnl)"=w635) -> ()  [unwired: 2 in, 2 out]
            n351 = local write "Stop Saving"(w637) -> ()
          }
          frame #1 {
            w638 = FALSE ("Fl. Triggered...")
            n352 = case shown="True" "Dump spot flow on?" {
              frame False {
              }
              frame True {
                n353 = property on="Sample Channel\nFlow" class="Bool (strict)"("Val(Sgnl)"=TRUE ("Stage Moving")) -> ()  [unwired: 2 in, 2 out]
              }
            }
            n354 = local write "Fl. Triggered..."(w638) -> ()
            n355 = local write "Tether"(w638) -> ()
            n356 = property on="Green Laser ON" class="Bool (strict)"("Val(Sgnl)"=w638) -> ()  [unwired: 2 in, 2 out]
            n357 = property on="Trap Pos. FB ON" class="Bool (strict)"("Val(Sgnl)"=w638) -> ()  [unwired: 2 in, 2 out]
            n358 = property on="Trap Trig. Fl." class="Bool (strict)"("Val(Sgnl)"=w638) -> ()  [unwired: 2 in, 2 out]
            n359 = property on="Fl. Triggered..." class="Bool (strict)"("Val(Sgnl)"=w638) -> ()  [unwired: 2 in, 2 out]
            n360 = property on="Dip for Protein" class="Bool (strict)"("Val(Sgnl)"=w638) -> ()  [unwired: 2 in, 2 out]
            n361 = property on="Pause dwell" class="Bool (strict)"("Val(Sgnl)"=w638) -> ()  [unwired: 2 in, 2 out]
          }
          frame #2 {
            n362 = property on="Trap Pos. FB Offset Factor" class="DigNum (strict)"("Val(Sgnl)"=i64 0 ("Value (Signaling)")) -> ()  [unwired: 2 in, 2 out]
          }
          frame #3 {
            n363 = local read "Saved Stage Positions"() -> (w647:dbl[][])
            n364 = local write "Stage Moving"(TRUE ("Stage Moving")) -> ()
            n365 = Array Subset(array=w647, index (row)=3 ("index"), length (row)=1 ("length"), index (col)=1 ("index"), length (col)=3 ("length")) -> (w652:dbl[][])
            n366 = Reshape Array(w652, 3 ("dimension size")) -> (w650:dbl[])
            n367 = Array To Cluster(array=w650) -> (cluster=w649:cluster{"[0]":dbl, "[1]":dbl, "[2]":dbl})
            n368 = call "Set Stage Position.vi"("Position"=w649, "error in"=w645, "VISA resource name in"=w646) -> ()  [unwired: 3 out]
          }
          frame #4 {
            w657 = FALSE ("Value (Signaling)")
            n369 = case shown="True" w656 {
              frame False {
              }
              frame True {
                n370 = property on="Sample Channel\nFlow" class="Bool (strict)"("Val(Sgnl)"=FALSE ("Stage Moving")) -> ()  [unwired: 2 in, 2 out]
              }
            }
            n371 = property on="Trap 1 (ON/OFF)" class="Bool (strict)"("Val(Sgnl)"=w657) -> ()  [unwired: 2 in, 2 out]
            n372 = property on="Trap 2 (ON/OFF)" class="Bool (strict)"("Val(Sgnl)"=w657) -> ()  [unwired: 2 in, 2 out]
            n373 = call <vilib>:"Beep.vi"() -> ()  [unwired: 3 in, 9 out]
          }
          frame #5 {
            n374 = property on="Move Cap. 2 (ADig Top)" class="Bool (strict)"("Val(Sgnl)"=TRUE ("Value (Signaling)")) -> ()  [unwired: 2 in, 2 out]
            n375 = property on="Tab Control" class="TabCtl (strict)"("Val(Sgnl)"=T39."Status" ("Value (Signaling)")) -> ()  [unwired: 2 in, 2 out]
          }
        }
      }
      event "Dip for Protein": Value Change {
        n376 = event-data() -> ()  [unwired: 1 in, 5 out]
        n377 = case shown="True" "Dip for Protein" {
          tunnel: w663 -> [_ w665]
          tunnel: w662 -> [_ w664]
          frame False {
          }
          frame True {
            n378 = while {
              tunnel: w665 -> [w676]
              tunnel: w664 -> [w675]
              i -> [w670]
              stop <- w672 stop-if-true
              n379 = Increment(x=w670) -> (x+1=→"Dip #":i32)
              n380 = flat-sequence {
                tunnel: w675 -> [w687]
                tunnel: w676 -> [w688]
                tunnel: [w688] -> w680
                tunnel: [w687] -> w679
                tunnel: [w681] -> w666
                tunnel: [w693] -> w674
                tunnel: [w694] -> w673
                tunnel: w680 -> [w695]
                tunnel: w679 -> [w696]
                tunnel: [w691] -> w667
                tunnel: w666 -> [w691]
                tunnel: [w704] -> w678
                tunnel: w674 -> [w704]
                tunnel: [w703] -> w677
                tunnel: w673 -> [w703]
                tunnel: [w700] -> w671
                tunnel: [w699] -> w668
                tunnel: w667 -> [w699]
                tunnel: w677 -> [w724]
                tunnel: w678 -> [w725]
                tunnel: w671 -> [w726]
                tunnel: w668 -> [w723]
                tunnel: [w782] -> w672
                frame #0 {
                  n381 = local read "Trap Pos. FB ON"() -> (w681:bool)
                  n382 = Compound Arithmetic op=AND("Flow ON\nduring dip?", "FB OFF when \nflow ON", w681) -> (w682:bool)
                  n383 = case shown="True" "Move trap \nbefore dip move?" {
                    frame False {
                    }
                    frame True {
                      n384 = property on="Trap Delta (MHz)" class="DigNum (strict)"("Val(Sgnl)"="Dipping Delta (MHz)") -> ()  [unwired: 2 in, 2 out]
                    }
                  }
                  n385 = property on="Green Laser ON" class="Bool (strict)"("Val(Sgnl)"="Green ON\nbefore dip?") -> ()  [unwired: 2 in, 2 out]
                  n386 = property on="Sample Channel\nFlow" class="Bool (strict)"("Val(Sgnl)"="Flow ON\nduring dip?") -> ()  [unwired: 2 in, 2 out]
                  n387 = case shown="True" w682 {
                    frame False {
                    }
                    frame True {
                      n388 = property on="Trap Pos. FB ON" class="Bool (strict)"("Val(Sgnl)"=FALSE ("Value (Signaling)")) -> ()  [unwired: 2 in, 2 out]
                    }
                  }
                }
                frame #1 {
                  n389 = local read "Saved Stage Positions"() -> (w698:dbl[][])
                  n390 = local write "Cancel dwell"(FALSE ("Cancel dwell")) -> ()
                  n391 = call "move to saved stage position.vi"("error in"=w696, "Stage VISA resource name in"=w695, "Position"="Dip Stage \nPosition", "Saved Stage Positions"=w698) -> ("VISA resource name out"=w693:refnum<visa-resource-name>, "error out"=w694:errorcluster)
                }
                frame #2 {
                  n392 = node-c288() -> (w702:T35)  [unwired: 4 in]
                  n393 = timed-loop {
                    timing: w702 -> [_]
                    timing-out: [_] -> w701
                    tunnel: [w708] -> w700
                    i -> [w705]
                    stop <- w709 stop-if-true
                    n394 = node-c288() -> ()  [unwired: 1 in, 1 out]
                    n395 = Greater Or Equal?(x=w705, y="Dip Duration (s)") -> (x >= y?=w717:bool)
                    n396 = local read "Dip for Protein"() -> (w710:bool)
                    n397 = local read "Dump Beads"() -> (w707:bool)
                    n398 = local read "Cancel dwell"() -> (w716:bool)
                    n399 = local read "Pause dwell"() -> (w713:bool)
                    n400 = Not(x=w710) -> (.not. x?=w715:bool)
                    n401 = Compound Arithmetic op=OR(w716, w717, w715) -> (w714:bool)
                    n402 = Select(t=FALSE, s=w713, f=w714) -> (s? t:f=w711:bool)
                    n403 = Not(x=w707) -> (.not. x?=w706:bool)
                    n404 = node-c288() -> ()  [unwired: 1 in, 1 out]
                    n405 = And(x=w710, y=w706) -> (x .and. y?=w708:bool)
                    n406 = Or(x=w711, y=w707) -> (x .or. y?=w709:bool)
                    "Dip Time (s)" <- w705
                  }
                  n407 = node-c288(w701) -> ()  [unwired: 1 out]
                }
                frame #3 {
                  n408 = case shown="True" w726 {
                    tunnel: w725 -> [_ w731]
                    tunnel: w724 -> [_ w730]
                    tunnel: w723 -> [_ w727]
                    frame False {
                    }
                    frame True {
                      n409 = flat-sequence {
                        tunnel: w730 -> [w735]
                        tunnel: w731 -> [w736]
                        tunnel: [w736] -> w729
                        tunnel: [w735] -> w728
                        tunnel: w727 -> [w732]
                        tunnel: w729 -> [w746]
                        tunnel: w728 -> [w745]
                        tunnel: w727 -> [w754]
                        frame #0 {
                          n410 = local read "Sample Channel\nFlow"() -> (w734:bool)
                          n411 = case shown="True" w734 {
                            tunnel: "Flow ON \nduring return\nfrom dip?" -> [w737 w740]
                            tunnel: w732 -> [_ w739]
                            frame False {
                              n412 = case shown="True" w737 {
                                frame False {
                                }
                                frame True {
                                n413 = property on="Sample Channel\nFlow" class="Bool (strict)"("Val(Sgnl)"=TRUE ("Value (Signaling)")) -> ()  [unwired: 2 in, 2 out]
                                }
                              }
                            }
                            frame True {
                              n414 = case shown="False" w740 {
                                tunnel: w739 -> [w741 _]
                                frame False {
                                n415 = property on="Trap Pos. FB ON" class="Bool (strict)"("Val(Sgnl)"=w741) -> ()  [unwired: 2 in, 2 out]
                                n416 = property on="Sample Channel\nFlow" class="Bool (strict)"("Val(Sgnl)"=FALSE ("Value (Signaling)")) -> ()  [unwired: 2 in, 2 out]
                                }
                                frame True {
                                }
                              }
                            }
                          }
                        }
                        frame #1 {
                          # "For turning on green laser before stage reaches lower spot"
                          n417 = case shown="True" "Green ON\nafter start\nreturn?" {
                            frame False {
                            }
                            frame True {
                              n418 = flat-sequence {
                                frame #0 {
                                n419 = Multiply(x="Green delay after \nstart return (s)", y=1000.0) -> (x*y=w751:dbl)
                                n420 = Wait (ms)(milliseconds to wait=w751) -> ()  [unwired: 1 out]
                                }
                                frame #1 {
                                n421 = property on="Green Laser ON" class="Bool (strict)"("Val(Sgnl)"=TRUE ("Value (Signaling)")) -> ()  [unwired: 2 in, 2 out]
                                }
                              }
                            }
                          }
                          n422 = local read "Saved Stage Positions"() -> (w749:dbl[][])
                          n423 = local write "Cancel dwell"(FALSE ("Cancel dwell")) -> ()
                          n424 = call "move to saved stage position.vi"("error in"=w745, "Stage VISA resource name in"=w746, "Position"="Return Stage \nPosition", "Saved Stage Positions"=w749) -> ("error out"=w747:errorcluster)  [unwired: 1 out]
                          n425 = local write "Stage Control Serial Error"(w747) -> ()
                        }
                        frame #2 {
                          n426 = property on="Trap Pos. FB ON" class="Bool (strict)"("Val(Sgnl)"=w754) -> ()  [unwired: 2 in, 2 out]
                          n427 = case shown="True" "Green ON \nafter return?" {
                            frame False {
                            }
                            frame True {
                              n428 = property on="Green Laser ON" class="Bool (strict)"("Val(Sgnl)"=TRUE ("Value (Signaling)")) -> ()  [unwired: 2 in, 2 out]
                            }
                          }
                          n429 = case shown="True" "Move trap after return?" {
                            frame False {
                            }
                            frame True {
                              n430 = property on="Trap Delta (MHz)" class="DigNum (strict)"("Val(Sgnl)"="Dip Trap Delta 2 (MHz)") -> ()  [unwired: 2 in, 2 out]
                            }
                          }
                          n431 = case shown="True" "Save data after return?" {
                            frame False {
                            }
                            frame True {
                              n432 = property on="Start Saving" class="Bool (strict)"("Val(Sgnl)"=TRUE ("Value (Signaling)")) -> ()  [unwired: 2 in, 2 out]
                            }
                          }
                          n433 = property on="Sample Channel\nFlow" class="Bool (strict)"("Val(Sgnl)"="Flow ON\nduring daq?") -> ()  [unwired: 2 in, 2 out]
                        }
                        frame #3 {
                          n434 = node-c288() -> (w763:T35)  [unwired: 4 in]
                          n435 = timed-loop {
                            timing: w763 -> [_]
                            timing-out: [_] -> w762
                            i -> [w764]
                            stop <- w766 stop-if-true
                            n436 = node-c288() -> ()  [unwired: 1 in, 1 out]
                            n437 = local read "Dump Beads"() -> (w765:bool)
                            n438 = Greater Or Equal?(x=w764, y="Dwell Duration (s)") -> (x >= y?=w771:bool)
                            n439 = local read "Dip for Protein"() -> (w768:bool)
                            n440 = Not(x=w768) -> (.not. x?=w767:bool)
                            n441 = Compound Arithmetic op=OR(w771, "Cancel dwell", w767) -> (w770:bool)
                            n442 = node-c288() -> ()  [unwired: 1 in, 1 out]
                            n443 = Select(t=FALSE, s="Pause dwell", f=w770) -> (s? t:f=w773:bool)
                            n444 = Or(x=w773, y=w765) -> (x .or. y?=w766:bool)
                            "Dwell Time (s)" <- w764
                          }
                          n445 = node-c288(w762) -> ()  [unwired: 1 out]
                        }
                      }
                    }
                  }
                }
                frame #4 {
                  n446 = local read "Dip for Protein"() -> (w783:bool)
                  n447 = local read "Dump Beads"() -> (w780:bool)
                  n448 = local write "Cancel dwell"(FALSE ("Cancel dwell")) -> ()
                  n449 = Not(x=w783) -> (.not. x?=w784:bool)
                  n450 = Not(x="Cont. Repeat Dipping?") -> (.not. x?=w786:bool)
                  n451 = Compound Arithmetic op=OR(w784, w786, w780) -> (w782:bool)
                }
              }
            }
          }
        }
      }
      event "Profile": Value Change {
        n452 = event-data() -> ()  [unwired: 1 in, 5 out]
        n453 = flat-sequence {
          tunnel: w795 -> [w798]
          tunnel: w794 -> [w806]
          tunnel: [w800] -> w793
          tunnel: [w799] -> w792
          tunnel: [w797] -> w790
          tunnel: [w796] -> w787
          tunnel: w793 -> [w813]
          tunnel: w792 -> [w812]
          tunnel: [w810] -> w791
          tunnel: w790 -> [w811]
          tunnel: [w809] -> w789
          tunnel: [w808] -> w788
          tunnel: w787 -> [w808]
          tunnel: w791 -> [w817]
          tunnel: w789 -> [w816]
          tunnel: w788 -> [w815]
          frame #0 {
            n454 = call "Read Stage Position.vi"("error in"=w806, "VISA resource name in"=w798) -> ("Current Position"=w796:cluster{dbl, dbl, dbl}, "error out"=w799:errorcluster, "VISA resource name out"=w797:refnum<visa-resource-name>)  [unwired: 1 out]
            "Current Position" <- w796
            n455 = local write "Stage Control Serial Error"(w799) -> ()
            n456 = Unbundle(w796) -> (w803:dbl, w805:dbl, w801:dbl)
            n457 = Add(x=w805, y="Y change (mm)") -> (x+y=w802:dbl)
            n458 = Bundle(w803, w802, w801) -> (w800:cluster{dbl, dbl, dbl})  [unwired: 1 in]
          }
          frame #1 {
            # "move to new position and start saving"